vi "SMain.vi"() -> ()   [LabVIEW 2011] (continued)
, 7358893750.0, 7365137500.0, 7371381250.0, 7377625000.0, 7383868750.0, 7390112500.0, 7396356250.0, 7402600000.0, 7408843750.0, 7415087500.0, 7421331250.0, 7427575000.0, 7433818750.0, 7440062500.0, 7446306250.0, 7452550000.0, 7458793750.0, 7465037500.0, 7471281250.0, 7477525000.0, 7483768750.0, 7490012500.0, 7496256250.0, 7502500000.0, 7508743750.0, 7514987500.0, 7521231250.0, 7527475000.0, 7533718750.0, 7539962500.0, 7546206250.0, 7552450000.0, 7558693750.0, 7564937500.0, 7571181250.0, 7577425000.0, 7583668750.0, 7589912500.0, 7596156250.0, 7602400000.0, 7608643750.0, 7614887500.0, 7621131250.0, 7627375000.0, 7633618750.0, 7639862500.0, 7646106250.0, 7652350000.0, 7658593750.0, 7664837500.0, 7671081250.0, 7677325000.0, 7683568750.0, 7689812500.0, 7696056250.0, 7702300000.0, 7708543750.0, 7714787500.0, 7721031250.0, 7727275000.0, 7733518750.0, 7739762500.0, 7746006250.0, 7752250000.0, 7758493750.0, 7764737500.0, 7770981250.0, 7777225000.0, 7783468750.0, 7789712500.0, 7795956250.0, 7802200000.0, 7808443750.0, 7814687500.0, 7820931250.0, 7827175000.0, 7833418750.0, 7839662500.0, 7845906250.0, 7852150000.0, 7858393750.0, 7864637500.0, 7870881250.0, 7877125000.0, 7883368750.0, 7889612500.0, 7895856250.0, 7902100000.0, 7908343750.0, 7914587500.0, 7920831250.0, 7927075000.0, 7933318750.0, 7939562500.0, 7945806250.0, 7952050000.0, 7958293750.0, 7964537500.0, 7970781250.0, 7977025000.0, 7983268750.0, 7989512500.0, 7995756250.0, 8002000000.0, 8008243750.0, 8014487500.0, 8020731250.0, 8026975000.0, 8033218750.0, 8039462500.0, 8045706250.0, 8051950000.0, 8058193750.0, 8064437500.0, 8070681250.0, 8076925000.0, 8083168750.0, 8089412500.0, 8095656250.0, 8101900000.0, 8108143750.0, 8114387500.0, 8120631250.0, 8126875000.0, 8133118750.0, 8139362500.0, 8145606250.0, 8151850000.0, 8158093750.0, 8164337500.0, 8170581250.0, 8176825000.0, 8183068750.0, 8189312500.0, 8195556250.0, 8201800000.0, 8208043750.0, 8214287500.0, 8220531250.0, 8226775000.0, 8233018750.0, 8239262500.0, 8245506250.0, 8251750000.0, 8257993750.0, 8264237500.0, 8270481250.0, 8276725000.0, 8282968750.0, 8289212500.0, 8295456250.0, 8301700000.0, 8307943750.0, 8314187500.0, 8320431250.0, 8326675000.0, 8332918750.0, 8339162500.0, 8345406250.0, 8351650000.0, 8357893750.0, 8364137500.0, 8370381250.0, 8376625000.0, 8382868750.0, 8389112500.0, 8395356250.0, 8401600000.0, 8407843750.0, 8414087500.0, 8420331250.0, 8426575000.0, 8432818750.0, 8439062500.0, 8445306250.0, 8451550000.0, 8457793750.0, 8464037500.0, 8470281250.0, 8476525000.0, 8482768750.0, 8489012500.0, 8495256250.0, 8501500000.0, 8507743750.0, 8513987500.0, 8520231250.0, 8526475000.0, 8532718750.0, 8538962500.0, 8545206250.0, 8551450000.0, 8557693750.0, 8563937500.0, 8570181250.0, 8576425000.0, 8582668750.0, 8588912500.0, 8595156250.0, 8601400000.0, 8607643750.0, 8613887500.0, 8620131250.0, 8626375000.0, 8632618750.0, 8638862500.0, 8645106250.0, 8651350000.0, 8657593750.0, 8663837500.0, 8670081250.0, 8676325000.0, 8682568750.0, 8688812500.0, 8695056250.0, 8701300000.0, 8707543750.0, 8713787500.0, 8720031250.0, 8726275000.0, 8732518750.0, 8738762500.0, 8745006250.0, 8751250000.0, 8757493750.0, 8763737500.0, 8769981250.0, 8776225000.0, 8782468750.0, 8788712500.0, 8794956250.0, 8801200000.0, 8807443750.0, 8813687500.0, 8819931250.0, 8826175000.0, 8832418750.0, 8838662500.0, 8844906250.0, 8851150000.0, 8857393750.0, 8863637500.0, 8869881250.0, 8876125000.0, 8882368750.0, 8888612500.0, 8894856250.0, 8901100000.0, 8907343750.0, 8913587500.0, 8919831250.0, 8926075000.0, 8932318750.0, 8938562500.0, 8944806250.0, 8951050000.0, 8957293750.0, 8963537500.0, 8969781250.0, 8976025000.0, 8982268750.0, 8988512500.0, 8994756250.0, 9001000000.0, 9007243750.0, 9013487500.0, 9019731250.0, 9025975000.0, 9032218750.0, 9038462500.0, 9044706250.0, 9050950000.0, 9057193750.0, 9063437500.0, 9069681250.0, 9075925000.0, 9082168750.0, 9088412500.0, 9094656250.0, 9100900000.0, 9107143750.0, 9113387500.0, 9119631250.0, 9125875000.0, 9132118750.0, 9138362500.0, 9144606250.0, 9150850000.0, 9157093750.0, 9163337500.0, 9169581250.0, 9175825000.0, 9182068750.0, 9188312500.0, 9194556250.0, 9200800000.0, 9207043750.0, 9213287500.0, 9219531250.0, 9225775000.0, 9232018750.0, 9238262500.0, 9244506250.0, 9250750000.0, 9256993750.0, 9263237500.0, 9269481250.0, 9275725000.0, 9281968750.0, 9288212500.0, 9294456250.0, 9300700000.0, 9306943750.0, 9313187500.0, 9319431250.0, 9325675000.0, 9331918750.0, 9338162500.0, 9344406250.0, 9350650000.0, 9356893750.0, 9363137500.0, 9369381250.0, 9375625000.0, 9381868750.0, 9388112500.0, 9394356250.0, 9400600000.0, 9406843750.0, 9413087500.0, 9419331250.0, 9425575000.0, 9431818750.0, 9438062500.0, 9444306250.0, 9450550000.0, 9456793750.0, 9463037500.0, 9469281250.0, 9475525000.0, 9481768750.0, 9488012500.0, 9494256250.0, 9500500000.0, 9506743750.0, 9512987500.0, 9519231250.0, 9525475000.0, 9531718750.0, 9537962500.0, 9544206250.0, 9550450000.0, 9556693750.0, 9562937500.0, 9569181250.0, 9575425000.0, 9581668750.0, 9587912500.0, 9594156250.0, 9600400000.0, 9606643750.0, 9612887500.0, 9619131250.0, 9625375000.0, 9631618750.0, 9637862500.0, 9644106250.0, 9650350000.0, 9656593750.0, 9662837500.0, 9669081250.0, 9675325000.0, 9681568750.0, 9687812500.0, 9694056250.0, 9700300000.0, 9706543750.0, 9712787500.0, 9719031250.0, 9725275000.0, 9731518750.0, 9737762500.0, 9744006250.0, 9750250000.0, 9756493750.0, 9762737500.0, 9768981250.0, 9775225000.0, 9781468750.0, 9787712500.0, 9793956250.0, 9800200000.0, 9806443750.0, 9812687500.0, 9818931250.0, 9825175000.0, 9831418750.0, 9837662500.0, 9843906250.0, 9850150000.0, 9856393750.0, 9862637500.0, 9868881250.0, 9875125000.0, 9881368750.0, 9887612500.0, 9893856250.0, 9900100000.0, 9906343750.0, 9912587500.0, 9918831250.0, 9925075000.0, 9931318750.0, 9937562500.0, 9943806250.0, 9950050000.0, 9956293750.0, 9962537500.0, 9968781250.0, 9975025000.0, 9981268750.0, 9987512500.0, 9993756250.0, 10000000000.0]
  out "Test Graph":refnum<vi>[](array[refnum])
  out "S-Pair Loop":i32=8
  out "S-Para Item List":string[](array[string])=["SDD21", "SDD11", "SCD22", "SCC11", "SCD21-SDD21", "ILD_15"]
  out "S Item Size":i32=6
  out "Spec Association Col No":string[](array[string])=["1", "2", "3", "4", "5", "6", "7"]
  out "Diff Test Item Name":string[](array[string])=["SDD21", "SDD11", "SCD22", "SCC11", "SCD21-SDD21", "NEXT", "ILD_15"]
  out "FEXT Pair Name":string[](array[string])=["TX2-RX1", "TX3-RX1", "TX4-RX1", "TX1-RX2", "TX3-RX2", "TX4-RX2", "TX1-RX3", "TX2-RX3", "TX4-RX3", "TX1-RX4", "TX2-RX4", "TX3-RX4"]
  out "NEXT Pair Name":string[](array[string])=["TX1-RX1", "TX2-RX1", "TX3-RX1", "TX4-RX1", "TX1-RX2", "TX2-RX2", "TX3-RX2", "TX4-RX2", "TX1-RX3", "TX2-RX3", "TX3-RX3", "TX4-RX3", "TX1-RX4", "TX2-RX4", "TX3-RX4", "TX4-RX4"]
  out "S-para Pair Name":string[](array[string])=["TX1", "RX1", "TX2", "RX2", "TX3", "RX3", "TX4", "RX4"]
  in  "Tab_System":enum32{"Test", "Report", "System", "Other"}(tab)=enum."Report"
  out "Pro Num":i64
  out "MO Num":i64
  out "UseAge":i64
  out "Used":i64
  in  "P/N:":string="L99QF015-SD-R"
  in  "S/N:":string="automatic sn"
  in  "MO:":string="E511D-160900761"
  out "proBar":dbl(slide) scale=0.0..100.0
  in  "Start Test":bool
  in  "Sample Description":string="Des:HW QSFP28 Passive Cable\rCable AWG:30\rLength:1000mm"
  in  "Result":string="Testing..."
  in  "Urgent Stop":bool
  in  "Test Status:":string="ILD_15将会采用与SDD21设定方式进行计算\n将生成精简的XML文件"
  in  "Temperature(℃)":string="163190001"
  in  "Relative Humidity(%)":string="163190001"
  in  "Fixture No":string="163190001"
  in  "Sample #":string="163190001"
  in  "Report No.":string="HF-163190001"
  in  "Applicant:":string
  in  "Approval:":u16(ring) items=["Chenhui Zeng", "Jet Shen"]
  in  "Tester:":u16(ring) items=["Wave Zhang", "Longjun Zhou", "Hui Pan", "Lindsay Gu", "Xiaoyue Xiang", "Fenglian Shi"]
  in  "Report Type:":u16(ring) items=["Excel", "Excel&PDF"]
  in  "Use Counts?":bool
  in  "By Channel?":bool
  out "Dem 2X":bool=TRUE
  in  "Local Database":bool
  in  "Demo":bool=TRUE
  in  "Manual":bool
  in  "Crosstalk  by Trace":bool
  in  "Adaptor:":enum16{"RS232 - IIC", "LUXSHARE - IIC"}(ring)=enum."LUXSHARE - IIC"
  in  "DAQ  Model:":T14(ring)
  in  "VNA VISA":refnum<visa-resource-name>="E5071C"
  in  "VNA Model:":enum16{"E5071C", "N5230A(C)", "N5224A"}(ring)
  in  "Port Type":u16(ring)=1
  in  "DAQ Device":u16(ring) items=["Dev1", "Dev2", "Dev3"]
  in  "Impedance Spec String":string="0.75@110@2@110;0.75@90@2@95"
  in  "VISA COM":refnum<visa-resource-name>="COM4"
  in  "Printer VISA":refnum<visa-resource-name>="COM4"
  in  "RS232 I2C VISA":refnum<visa-resource-name>="COM3"
  in  "save config":bool
  in  "打印模式":enum16{"IT Print", "EE Print"}(ring)=enum."EE Print" caption="Print Mode"
  in  "RS232 I2C Counts":refnum<visa-resource-name>="COM3"
  in  "Auto Count:":bool
  in  "Fast Print":bool=TRUE
  in  "测试模式":u16(ring) items=["正常", "调机", "校正"]
  in  "制程条码":bool
  in  "SN Keep":bool
  in  "Pre Check":bool
  in  "Type":u16(ring) items=["SFP+", "QSFP28"]
  in  "preStation":string="A0075"
  out "Current Testing Label/当前测试条码":string
  out "ratio":dbl format="%#_g%%"
  out "Total":dbl
  out "Failed":dbl
  out "Passed":dbl
  in  "线别":u16(ring) items=["XT026", "XT027", "XT028", "other"]
  in  "sampleNo":u16(ring) items=["0.009", "014-30", "11", "125553", "15669", "2018     8     20", "2018   8  7", "233665", "741", "755", "785587", "7896987", "a", "L021254", "L9956255", "L99901", "L99SF014-SD-H校准", "L99SF025-SD-R", "LDUQF007-18.6.22", "校准"]
  in  "Tab_Graph":T15(tab)
  out "PASS":cluster{"Horz Time array":dbl[], "Y":dbl[]}[](graph) caption="SDD21"
  out "PASS":cluster{"Horz Time array":dbl[], "Y":dbl[]}[](graph) caption="SDD11"
  out "Test Graph3":cluster{"Horz Time array":dbl[], "Y":dbl[]}[](graph) caption="SCC11"
  out "Test Graph4":cluster{"Horz Time array":dbl[], "Y":dbl[]}[](graph) caption="SCD21-SDD21"
  out "Test Graph5":cluster{"Horz Time array":dbl[], "Y":dbl[]}[](graph) caption="ILD"
  out "Test Graph6":cluster{"Horz Time array":dbl[], "Y":dbl[]}[](graph) caption="ILD"
  out "Test Graph7":cluster{"Horz Time array":dbl[], "Y":dbl[]}[](graph) caption="SCD21-SDD21"
  out "Test Graph8":cluster{"Horz Time array":dbl[], "Y":dbl[]}[](graph) caption="Pskew"
  out "TDD11 Graph":cluster{"Horz Time array":dbl[], "Y":dbl[]}[](graph) caption="TDD11"
  out "TDD22 Graph":cluster{"Horz Time array":dbl[], "Y":dbl[]}[](graph) caption="TDD22"
  out "TCC11":cluster{"Horz Time array":dbl[], "Y":dbl[]}[](graph) caption="TDD22"
  out "TCC22":cluster{"Horz Time array":dbl[], "Y":dbl[]}[](graph) caption="TDD22"
  out "Delay":cluster{"Horz Time array":dbl[], "Y":dbl[]}[](graph) caption="TDD22"
  out "Next":cluster{"Horz Time array":dbl[], "Y":dbl[]}[](graph) caption="NEXT"
  out "Test Graph10":cluster{"Horz Time array":dbl[], "Y":dbl[]}[](graph) caption="FEXT_TX2-RX1"
  out "MDFEXT":cluster{"Horz Time array":dbl[], "Y":dbl[]}[](graph) caption="FEXT_TX2-RX1"
  out "MDNEXT":cluster{"Horz Time array":dbl[], "Y":dbl[]}[](graph) caption="FEXT_TX2-RX1"
  # "HPTS Of  VNA Automatic Measurement System"
  # "Rev: 3.0.0.0\n18/06/07"
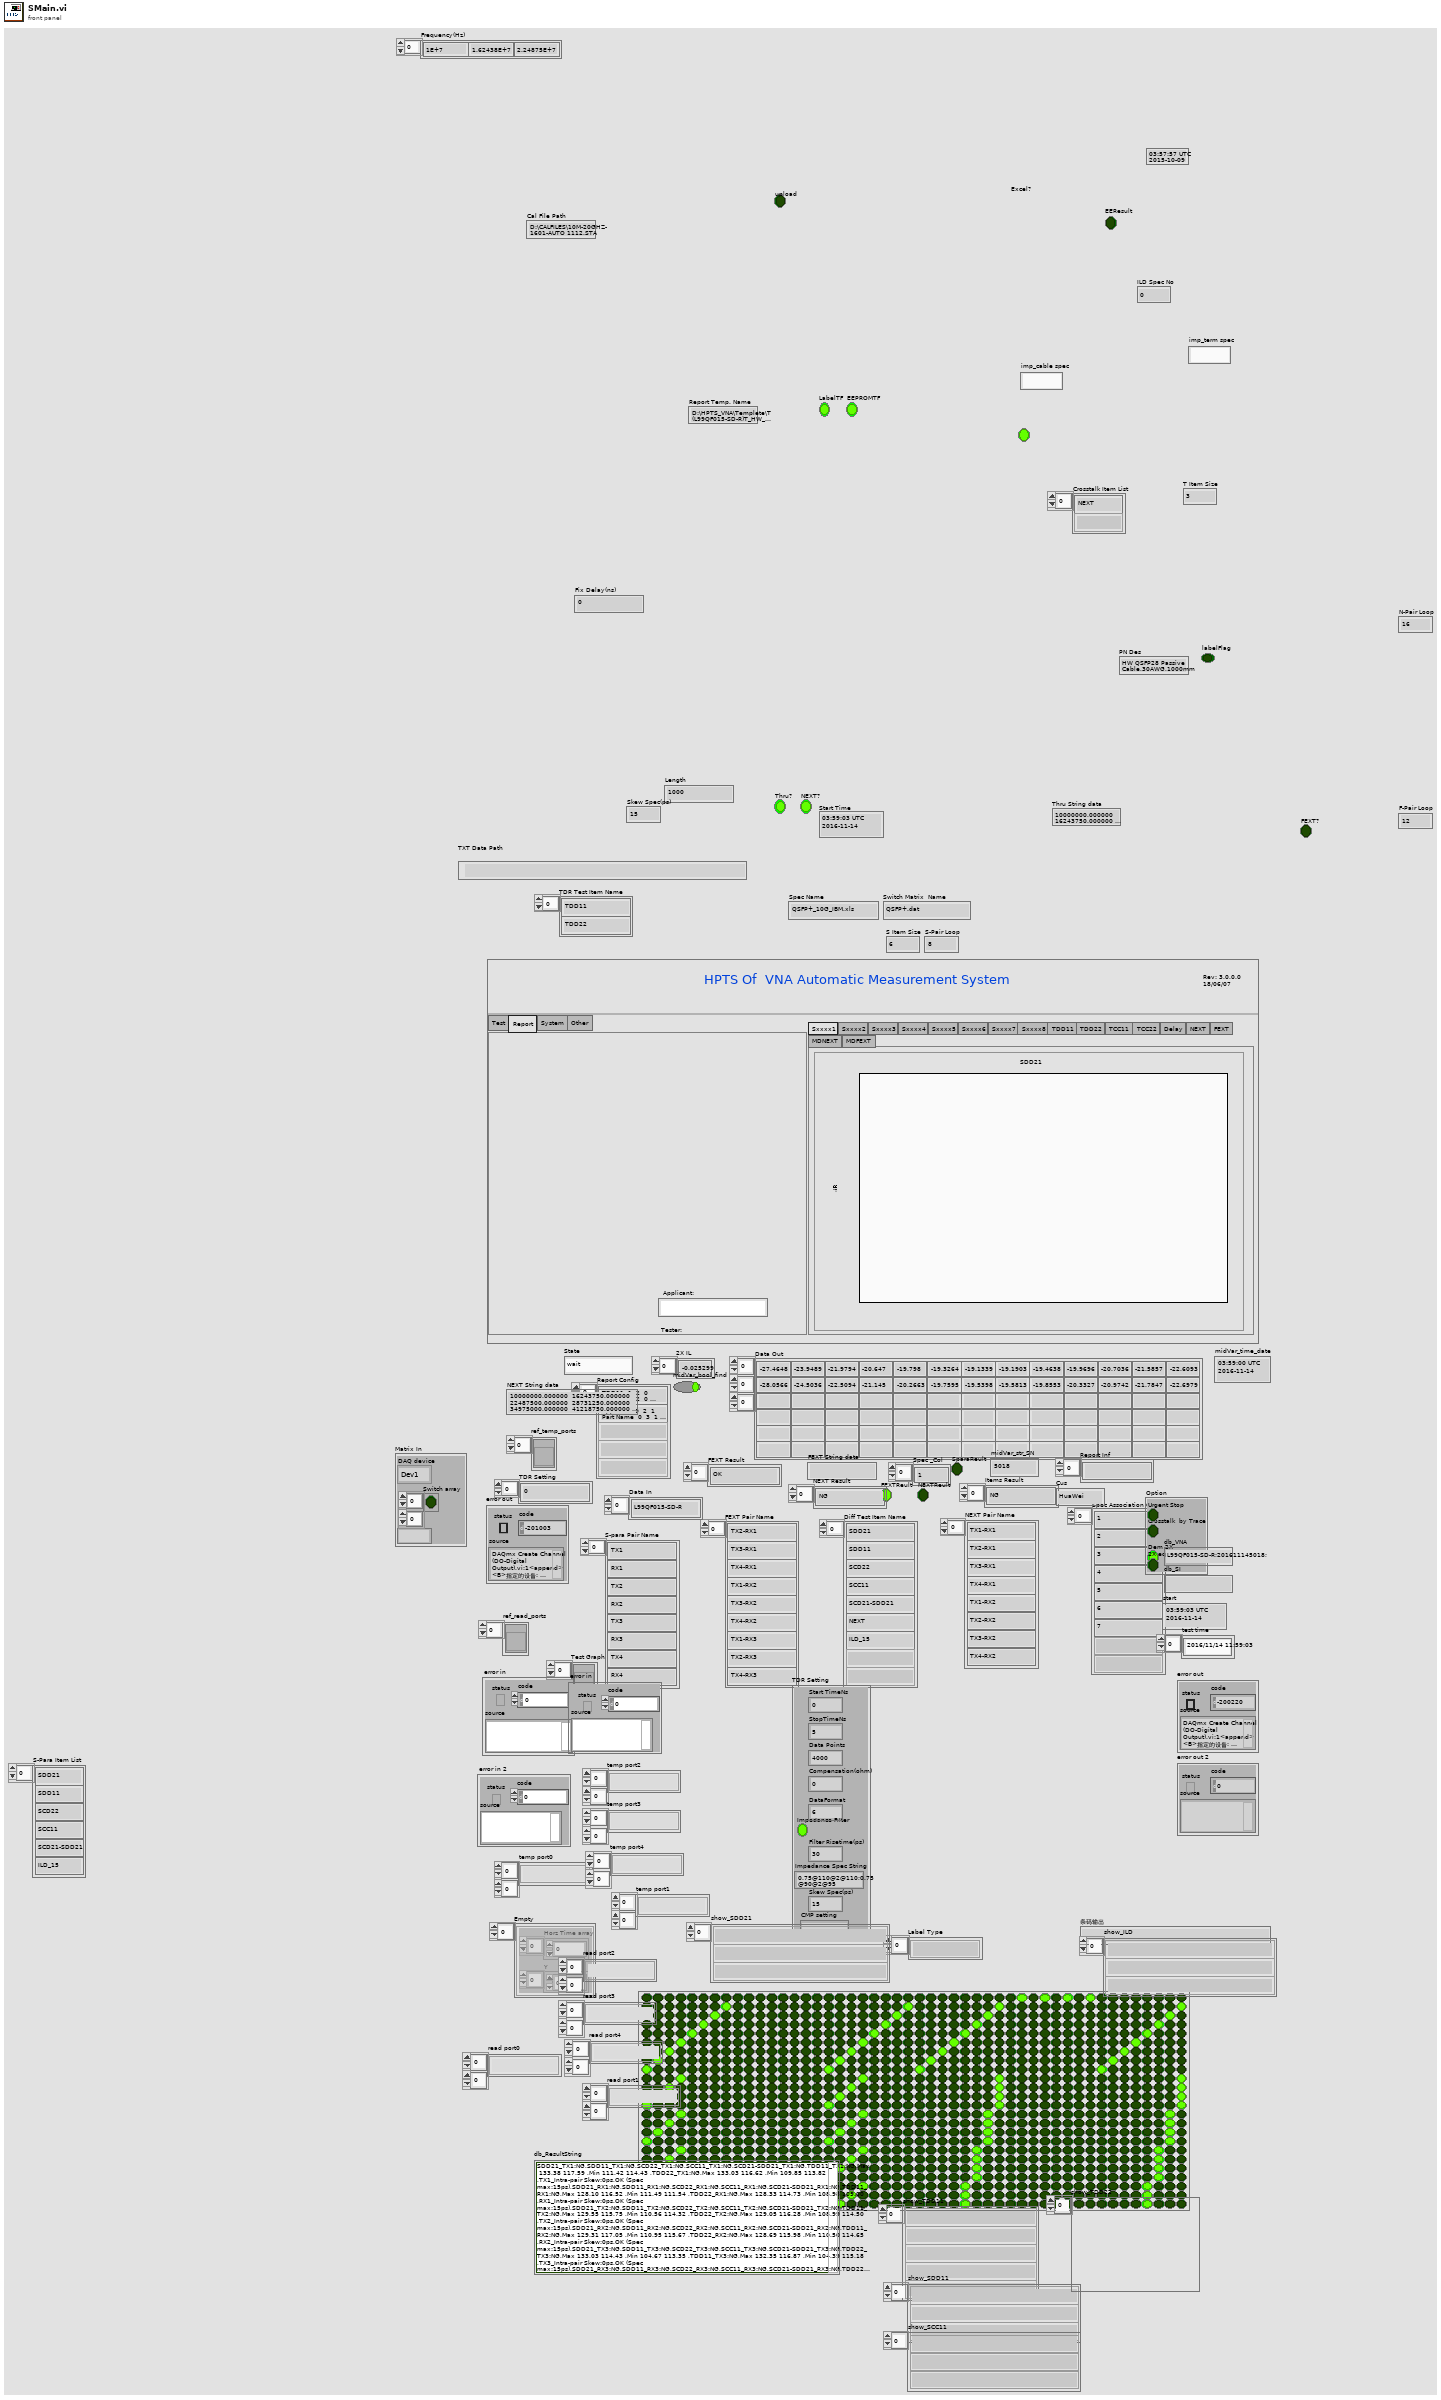
[diagram p1: front panel]
types:
  T1 = typedef "UploadPara.ctl" = cluster{"NetCmdHW":string, "NetPathHW":string, "NetCmdCompress":string, "NetPathCompress1":string, "NetPathCompress2":string, "AlarmDisplay":string, "Synchronous":string, "NetTemppath":string, "NetLocalpath":string}
  T2 = typedef "cluResult.ctl" = cluster{"itemResult":string[], "itemName":string[]}
  T3 = typedef "singleTestParameter.ctl" = cluster{"itemName":string, "testPair":dbl, "chartDisplay?":bool, "spec":cluster{"upper limit":cluster{"dx":dbl[], "dy":dbl[]}, "lowwer limit":cluster{"dx":dbl[], "dy":dbl[]}}, "smooth":cluster{"smooth?":bool, "smoothPoints":dbl}, "Compensation(ohm)":dbl, "Filter Risetime(ps)":dbl, "singlePoint":string[], "offset":dbl[]}
  T4 = typedef "informationIn.ctl" = cluster{"Sample PN: ":string, "SampleSN:":string, "Sparam Test Item":string[], "S-para Pair Name":string[], "Length":string, "Diff Test Item Name":string[], "Diff Test Item Name smooth":string[], "smooth point":dbl, "limitSpec":string[][], "switchIndexOffset":i32, "testType":enum16{"Loss", "Next", "Fext"}, "pairStartIndex":i32, "DAQ  Model:":enum16{"NI PCI-6509", "LX MCU", "LX MCU_40G", "LX MCU_40G_HuaWei"}, "VISA COM":refnum<visa-resource-name>, "Matrix  In":bool[][]}
  T5 = cluster{"Tab_Graph":refnum<vi>, "Test Graph":refnum<vi>[], "Test Status:":refnum<vi>, "db_ResultString":refnum<vi>}
  T6 = cluster{"Start TimeNs":dbl, "StopTimeNs":dbl, "Data Points":i32, "Compensation(ohm)":dbl, "DataFormat":i16, "Impedance Filter":bool, "Filter Risetime(ps)":dbl, "Impedance Spec String":string, "Skew Spec(ps)":i32, "CMP Setting":string}[]
  T7 = cluster{"start":i32, "length":i32, "p":i32, "H/L":bool}[]
  T8 = cluster{"Server":string, "DB":string, "PSW":string, "User":string}
  T9 = cluster{"auto get refer point":bool, "width1":i32, "width2":i32, "show_TDD11":string[], "show_TDD22":string[], "test time":string[], "show_impspec":string[], "TestResult":bool[], "FileName":string, "FileVersion":string}
  T10 = cluster{"Start TimeNs":dbl, "StopTimeNs":dbl, "Data Points":i32, "Compensation(ohm)":dbl, "DataFormat":i16, "Impedance Filter":bool, "Filter Risetime(ps)":dbl, "Impedance Spec String":string, "Skew Spec(ps)":i32, "CMP Setting":string}
  T11 = cluster{"Urgent Stop":bool, "Crosstalk  by Trace":bool, "Dem 2X":bool, "2X equalize ":bool}
  T12 = cluster{"Start TimeNs":dbl, "StopTimeNs":dbl, "Data Points":i32, "Compensation(ohm)":dbl, "DataFormat":i16, "Impedance Filter":bool, "Filter Risetime(ps)":dbl, "Impedance Spec String":string, "Skew Spec(ps)":i32, "CMP setting":string}
  T13 = cluster{"DAQ device":enum16{"Dev1", "Dev2", "Dev3"}, "Switch array ":bool[][], i32}
  T14 = enum16{"NI PCI-6509", "LX MCU", "LX MCU_40G", "LX MCU_40G_HuaWei"}
  T15 = enum32{"Sxxxx1", "Sxxxx2", "Sxxxx3", "Sxxxx4", "Sxxxx5", "Sxxxx6", "Sxxxx7", "Sxxxx8", "TDD11", "TDD22", "TCC11", "TCC22", "Delay", "NEXT", "FEXT", "MDNEXT", "MDFEXT"}
  T16 = enum16{"Standard Report", "HTML", "Word", "Excel"}
  T17 = enum8{"Enabled", "Disabled", "Disabled and Grayed Out"}
  T18 = typedef "HW_xml.ctl" = cluster{"FileVersion":string, "FileName":string, "test time":string[], "original Path":path, "show_impspec":string[], "usedSN":string, "show_Terminal Point":dbl[], "show_Cable Point":dbl[], "sSpec":T3[], "resultCluster":T2, "customerPN":string}
  T19 = enum32{"invalid app kind", "Development System", "Run Time System", "Student Edition", "Embedded LabVIEW", "Evaluation", "Custom"}
  T20 = cluster{"Urgent Stop":bool, "Crosstalk  by Trace":bool, "Dem 2X":bool, "2x equalize ":bool}
  T21 = cluster{"Demo":bool, "Manual":bool, "Urgent Stop":bool}
  T22 = cluster{"DAQ Device":u16, "Switch array ":bool[][], i32}
  T23 = cluster{"Start TimeNs 2":dbl, "StopTimeNs 2":dbl, "Data Points 2":i32, "Compensation(ohm) 2":dbl, "DataFormat":i16, bool, "Filter Risetime(ps) 2":dbl, "Impedance Spec String 2":string, "Skew Spec(ps) 2":i32, string}
  T24 = cluster{"DAQ Device":u16, "Switch array ":bool[][], "S-Pair Loop":i32}
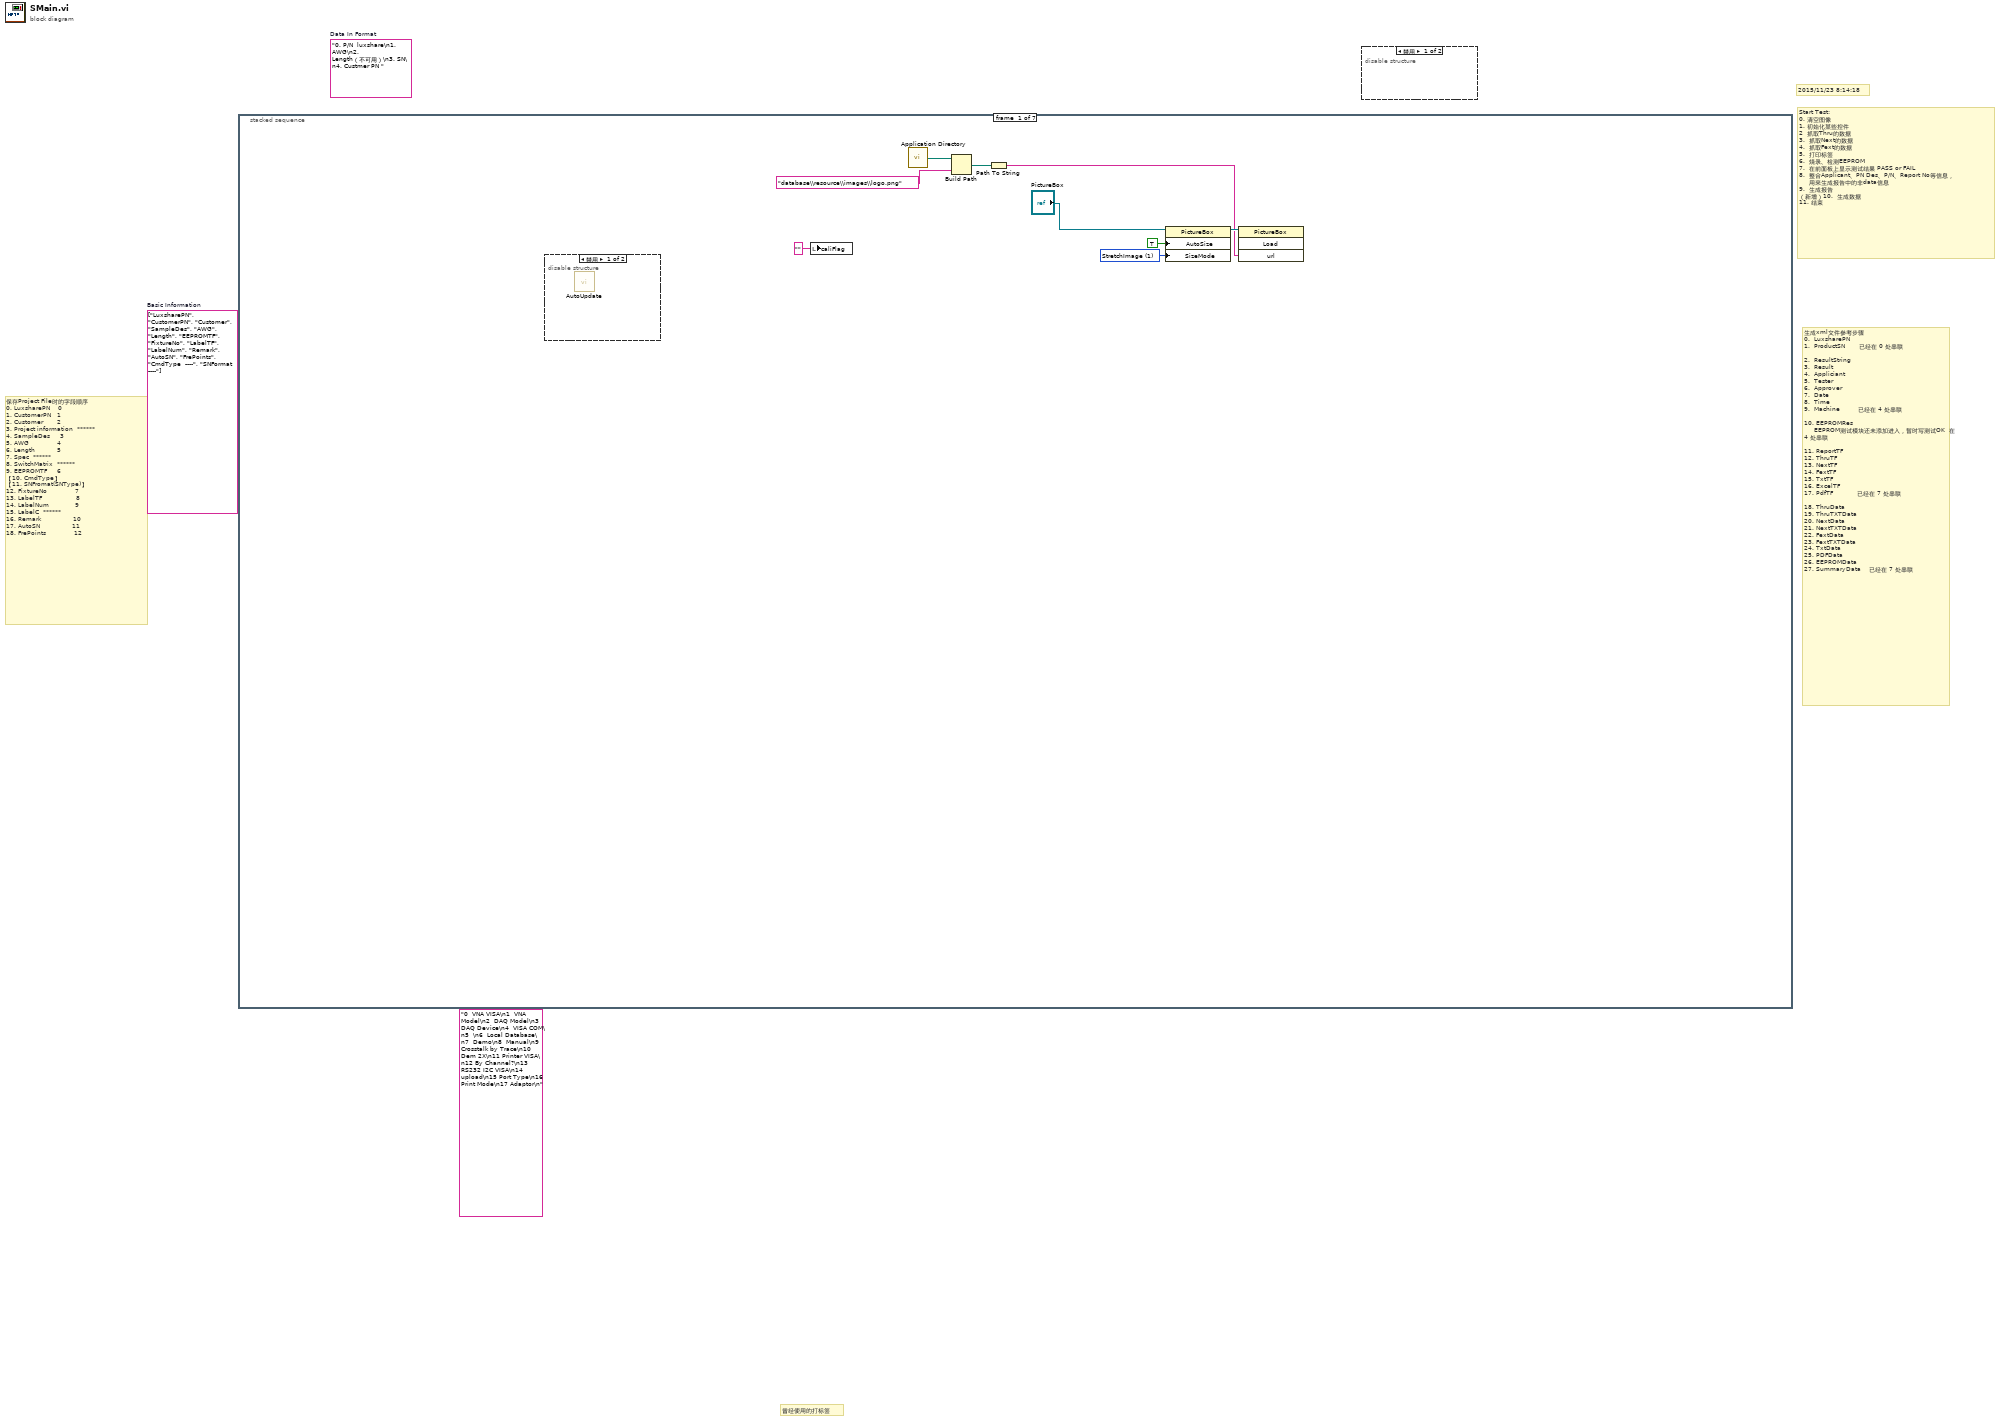
[diagram p0: block diagram]
diagram:
  (unwired) "0  VNA VISA\n1  VNA Model\n2  DAQ Model\n3  DAQ Device\n4  VISA COM\n5  \n6  Local Database\n7  Demo\n8  Manual\n9  Crosstalk by Trace\n10 Dem 2X\n11 Printer VISA\n12 By Channel?\n13 RS232 I2C VISA\n14 upload\n15 Port Type\n16 Print Mode\n17 Adaptor\n"
  (unwired) string[] ["LuxsharePN", "CustomerPN", "Customer", "SampleDes", "AWG", "Length", "EEPROMTF", "FixtureNo", "LabelTF", "LabelNum", "Remark", "AutoSN", "FrePoints", "CmdType  ----", "SNFormat ----"]  # Basic Information
  (unwired) "0. P/N  luxshare\n1. AWG\n2. Length（不可用）\n3. SN\n4. Custmer PN "  # Data In Format
  # "曾经使用的打标签"
  # "保存Project File时的字段顺序\n0. LuxsharePN    0 \n1. CustomerPN   1\n2. Customer       2\n3. Project information  ****** \n4. SampleDes     3\n5. AWG              4\n6. Length           5\n7. Spec  ******\n8. SwitchMatrix  ******  \n9. EEPROMTF     6\n【10. CmdType】           \n【11. SNFromat(SNType)】   \n12. FixtureNo              7\n13. LabelTF                 8\n14. LabelNum             9\n15. LabelC  ******\n16. Remark                10\n17. AutoSN                11\n18. FrePoints              12"
  # "2015/11/23 8:14:18"
  # "生成xml文件参考步骤\n0.  LuxsharePN\n1.  ProductSN       已经在 0 处串联\n\n2.  ResultString     \n3.  Result             \n4.  Appliciant\n5.  Tester\n6.  Approver\n7.  Date \n8.  Time\n9.  Machine         已经在 4 处串联\n\n10. EEPROMRes   \n     EEPROM测试模块还未添加进入，暂时写测试OK  在 4 处串联\n\n11. ReportTF\n12. ThruTF\n13. NextTF\n14. FextTF\n15. TxtTF\n16. ExcelTF\n17. PdfTF            已经在 7 处串联\n\n18. ThruData\n19. ThruTXTData\n20. NextData\n21. NextTXTData\n22. FextData\n23. FextTXTData\n24. TxtData\n25. PDFData\n26. EEPROMData\n27. SummaryData    已经在 7 处串联"
  # "Start Test:\n0. 清空图像\n1. 初始化某些控件 \n2  抓取Thru的数据\n3.  抓取Next的数据\n4.  抓取Fext的数据\n5.  打印标签\n6.  烧录、检测EEPROM\n7.  在前面板上显示测试结果 PASS or FAIL\n8.  整合Applicant、PN Des、P/N、Report No等信息，\n     用来生成报告中的非data信息\n9.  生成报告\n（新增）10.  生成数据 \n11. 结束"
  n1 = stacked-sequence {
    frame #0 {
      w5 = 1 items=["Normal", "StretchImage", "AutoSize", "CenterImage", "Zoom"] ("SizeMode")
      n2 = disable-structure shown="禁用" {
        frame Disabled {
          n3 = call "AutoUpdate.vi"() -> ()  [unwired: 8 in, 2 out]
        }
        frame Enabled {
        }
      }
      n4 = local write "caliFlag"("" ("caliFlag")) -> ()
      n5 = call <vilib>:"Application Directory.vi"() -> ("Application Directory"=w4:path)
      n6 = Build Path(base path=w4, name or relative path="database\\resource\\images\\logo.png" ("名称或相对路径")) -> (appended path=w2:path)
      n7 = Path To String(path=w2) -> (string=w1:string)
      n8 = property class="PictureBox"(reference="PictureBox", "AutoSize"=TRUE, "SizeMode"=w5) -> (reference out=w7:refnum<k24>)  [unwired: 1 in, 1 out]
      n9 = invoke class="PictureBox" method="Load"(reference=w7, "url"=w1) -> ()  [unwired: 2 in, 4 out]
    }
    frame #1 {
      # "中间变量"
      n10 = property class="App"() -> ("App.Kind"=w10:T19)  [unwired: 2 in, 2 out]
      n11 = case shown="\"Run Time System\", 默认" w10 {
        frame "Run Time System", Default {
          w12 = ".exe" ("正则表达式")
          n12 = Current VI's Path() -> (path=w15:path)
          n13 = Path To String(path=w15) -> (string=w14:string)
          n14 = xnode "匹配正则表达式"("输入字符串"=w14, "正则表达式"=w12) -> ("匹配之前"=w13:string)  [unwired: 4 in, 4 out]
          n15 = call <vilib>:"Application Directory.vi"() -> ("Application Directory"=w25:path)
          n16 = Build Path(base path=w25, name or relative path="AutoUpdate.xml" ("名称或相对路径")) -> (appended path=w23:path)
          n17 = Concatenate Strings(w13, w12) -> (→"FileName":string)
          n18 = call "xmlConfigRead.vi"("path to XML document"=w23, "XPath expression"="//@Ver") -> ("OutParaArray"=w22:string[])  [unwired: 2 out]
          n19 = Index Array(array=w22, index=4 ("索引")) -> (element=w17:string)
          n20 = call <vilib>:"Trim Whitespace.vi"("string"=w17) -> ("trimmed string"=w20:string)  [unwired: 1 in]
          n21 = String Length(string=w20) -> (length=w19:i32)
          n22 = Equal To 0?(x=w19) -> (x = 0?=w18:bool)
          n23 = case shown="假" w18 {
            tunnel: w17 -> [w138 _]
            tunnel: [w138 "9.9.9.9" ("node text")] -> w16
            frame False {
            }
            frame True {
              n24 = One Button Dialog(message="读取AutoUpdate.xml失败，使用程序默认版本号9.9.9.9" ("消息")) -> ()  [unwired: 1 in, 1 out]
            }
          }
          "FileVersion" <- w16
        }
        frame "Development System" {
          w141 = "DevelopmentSystem" ("FileName")
          n25 = property on="FileName" class="Str"("Value"=w141) -> ()  [unwired: 2 in, 2 out]
          n26 = property on="FileVersion" class="Str"("Value"=w141) -> ()  [unwired: 2 in, 2 out]
        }
      }
    }
    frame #2 {
      w160 = u16 0 items=["Excel", "Excel&PDF"] ("Report Type:")
      w161 = FALSE ("可见")
      w157 = FALSE ("Manual")
      w202 = 2 ("索引")
      w169 = "" ("Sample Description")
      w204 = 0 ("索引")
      n27 = control-ref of="proBar"() -> (→"proBar_ref":refnum<vi>)
      n28 = local write "preStation"("" ("preStation")) -> ()
      n29 = local write "Excel?"(FALSE ("Local Database")) -> ()
      n30 = local write "AutoSN"(FALSE ("AutoSN")) -> ()
      n31 = local write "P/N:"(w169) -> ()
      n32 = property on="Sample Description" class="Str"("Value"="" ("Sample Description"), "Visible"=FALSE ("可见")) -> ()  [unwired: 2 in, 2 out]
      n33 = property on="Tab_System" class="TabCtl (严格)"("Value"=w204) -> ()  [unwired: 2 in, 2 out]
      n34 = property on="Tab_Graph" class="TabCtl (严格)"("Value"=w204) -> ()  [unwired: 2 in, 2 out]
      n35 = property on="Start Test" class="Bool"("DisabledEnum"=w202) -> ()  [unwired: 2 in, 2 out]
      n36 = property on="VNA Initial" class="Bool"("DisabledEnum"=w202) -> ()  [unwired: 2 in, 2 out]
      n37 = local write "Impedance Spec String"(w169) -> ()
      n38 = control-ref of="Delay"() -> (w142:refnum<vi>)
      n39 = control-ref of="TCC11"() -> (w144:refnum<vi>)
      n40 = control-ref of="TCC22"() -> (w143:refnum<vi>)
      n41 = local write "State"("wait" ("state")) -> ()
      n42 = control-ref of="MDNEXT"() -> (w145:refnum<vi>)
      n43 = control-ref of="PASS"() -> (w214:refnum<vi>)
      n44 = control-ref of="PASS"() -> (w213:refnum<vi>)
      n45 = control-ref of="Test Graph3"() -> (w212:refnum<vi>)
      n46 = control-ref of="Test Graph4"() -> (w211:refnum<vi>)
      n47 = control-ref of="Test Graph5"() -> (w210:refnum<vi>)
      n48 = control-ref of="Test Graph6"() -> (w209:refnum<vi>)
      n49 = control-ref of="Test Graph7"() -> (w208:refnum<vi>)
      n50 = control-ref of="Test Graph8"() -> (w207:refnum<vi>)
      n51 = control-ref of="TDD11 Graph"() -> (w194:refnum<vi>)
      n52 = control-ref of="TDD22 Graph"() -> (w193:refnum<vi>)
      n53 = control-ref of="Next"() -> (w192:refnum<vi>)
      n54 = control-ref of="Test Graph10"() -> (w191:refnum<vi>)
      n55 = control-ref of="MDFEXT"() -> (w146:refnum<vi>)
      n56 = local write "Current Testing Label/当前测试条码"("") -> ()
      n57 = Build Array(w214, w213, w212, w211, w210, w209, w208, w207, w194, w193, w144, w143, w142, w192, w191, w146, w145) -> (w206:refnum<vi>[])
      "Test Graph" <- w206
      n58 = property on="Result" class="Str"("Visible"=FALSE ("可见"), "Value"="Testing..." ("Result"), "DisabledEnum"=1, "Text.BGColor"=u32 16777216) -> ()  [unwired: 2 in, 2 out]
      n59 = local write "Demo"(w157) -> ()
      n60 = local write "Dem 2X"(w157) -> ()
      n61 = local write "Manual"(w157) -> ()
      n62 = local write "Excel?"(w157) -> ()
      n63 = property on="Urgent Stop" class="Bool (严格)"("DisabledEnum"=0 ("索引")) -> ()  [unwired: 2 in, 2 out]
      n64 = property on="Report Type:" class="Ring (严格)"("Value"=w160) -> ()  [unwired: 2 in, 2 out]
      n65 = property on="Start Page" class="DigNum (严格)"("Visible"=w161) -> ()  [unwired: 2 in, 2 out]
      n66 = property on="End Page" class="DigNum (严格)"("Visible"=w161) -> ()  [unwired: 2 in, 2 out]
      n67 = local write "Local Database"(w157) -> ()
      n68 = local write "Auto Count:"(w157) -> ()
      n69 = local write "Crosstalk  by Trace"(w157) -> ()
      n70 = local write "Urgent Stop"(w157) -> ()
      n71 = for {
        tunnel: w206 -> [w248] mode=indexing
        tunnel: "Empty" -> [w247]
        n72 = property class="XYGraph (严格)"(reference=w248, "Value"=w247, "Caption.Visible"=FALSE ("标题.可见")) -> ()  [unwired: 1 in, 2 out]
      }
      n73 = call "运行批处理.vi"() -> ()  [unwired: 12 in]
      n74 = local write "Use Counts?"(TRUE ("Use Counts?")) -> ()
      n75 = local read "VISA COM"() -> (w168:refnum<visa-resource-name>)
      n76 = local read "DAQ Device"() -> (w166:u16)
      n77 = stacked-sequence {
        frame #0 {
          n78 = control-ref of="temp port0"() -> (w220:refnum<vi>)
          n79 = control-ref of="temp port1"() -> (w219:refnum<vi>)
          n80 = control-ref of="temp port2"() -> (w218:refnum<vi>)
          n81 = control-ref of="temp port3"() -> (w217:refnum<vi>)
          n82 = control-ref of="temp port4"() -> (w216:refnum<vi>)
          n83 = Build Array(w220, w219, w218, w217, w216) -> (→"ref_temp_ports":refnum<vi>[])
        }
        frame #1 {
          n84 = control-ref of="read port0"() -> (w226:refnum<vi>)
          n85 = control-ref of="read port1"() -> (w225:refnum<vi>)
          n86 = control-ref of="read port2"() -> (w224:refnum<vi>)
          n87 = control-ref of="read port3"() -> (w223:refnum<vi>)
          n88 = control-ref of="read port4"() -> (w222:refnum<vi>)
          n89 = Build Array(w226, w225, w224, w223, w222) -> (→"ref_read_ports":refnum<vi>[])
        }
      }
      n90 = local read "Manual"() -> (w164:bool)
      n91 = local read "DAQ  Model:"() -> (w167:T14)
      n92 = local read "Demo"() -> (w163:bool)
      n93 = Format Date/Time String(time format string (%c)="%#j") -> (date/time string=w197:string)  [unwired: 2 in]
      n94 = String Length(string=w197) -> (length=w198:i32)
      n95 = Or(x=w164, y=w163) -> (x .or. y?=w165:bool)
      n96 = call <vilib>:"Application Directory.vi"() -> ("Application Directory"=w181:path)
      n97 = case shown="2" w198 {
        tunnel: w197 -> [w240 w244 w245]
        tunnel: [w239 w243 w245] -> w196
        frame 1, Default {
          n98 = Concatenate Strings("00" ("字符串"), w240) -> (w239:string)
        }
        frame 2 {
          n99 = Concatenate Strings("0" ("字符串"), w244) -> (w243:string)
        }
        frame 3 {
        }
      }
      n100 = Build Path(base path=w181, name or relative path="database\\inf.txt" ("名称或相对路径")) -> (appended path=w179:path)
      n101 = case shown="假" w165 {
        tunnel: w166 -> [w229 _]
        tunnel: w167 -> [w228 _]
        tunnel: w168 -> [w227 _]
        frame False {
          n102 = case shown="\"LX MCU\"" w228 {
            tunnel: w229 -> [w234 _ _]
            tunnel: w227 -> [_ w236 w238]
            frame "NI PCI-6509", Default {
              n103 = local read "Switch array"() -> (w232:bool[][])
              n104 = call "6509 simple.vi"("error in"="error in", "index (row)"=i8 79, "array input: P0-P1-P2-P3-P4-P5"=w232, "DAQ device"=w234) -> ("error out"=→"error out":errorcluster)  [unwired: 3 in]
            }
            frame "LX MCU" {
              w235 = u16 1 items=["Testing", "Close All"] ("Function")
              n105 = call "MCU Switch Control.vi"("Function"=w235, "VISA"=w236) -> ()  [unwired: 9 in, 1 out]
            }
            frame "LX MCU_40G" {
              w237 = u16 1 items=["Testing", "Close All"] ("Function")
              n106 = call "40G MCU Switch Control.vi"("Function"=w237, "VISA"=w238) -> ()  [unwired: 9 in, 1 out]
            }
          }
        }
        frame True {
        }
      }
      n107 = call-poly <vilib>:"Read From Spreadsheet File.vi"("file path (dialog if empty)"=w179) -> ("all rows"=w178:string[][])  [unwired: 6 in, 4 out]
      n108 = Delete From Array(array=w178, index (row)=0 ("索引 (行)")) -> (array with subset deleted=w176:string[][])  [unwired: 2 in, 1 out]
      n109 = Format Date/Time String(time format string (%c)="%#y") -> (date/time string=w201:string)  [unwired: 2 in]
      n110 = Index Array(array=w176, index (col) #1=6 ("禁用的索引 (列)"), index (col) #2=7 ("索引 (列)")) -> (element #1=w173:string[], element #2=w172:string[])  [unwired: 2 in]
      n111 = Concatenate Strings(w201, w196, "0001" ("字符串")) -> (w182:string)
      n112 = call "Delete empty element from array.vi"("Array In"=w173) -> ("Array out"=w171:string[])  [unwired: 26 in]
      n113 = local write "Sample #"(w182) -> ()
      n114 = call "Delete empty element from array.vi"("Array In"=w172) -> ("Array out"=w170:string[])  [unwired: 26 in]
      n115 = local write "S/N:"(w182) -> ()
      n116 = Concatenate Strings("HF-" ("字符串"), w182) -> (w184:string)
      n117 = property on="Approval:" class="Ring (严格)"("Strings []"=w170) -> ()  [unwired: 2 in, 2 out]
      n118 = property on="Tester:" class="Ring (严格)"("Strings []"=w171) -> ()  [unwired: 2 in, 2 out]
      n119 = local write "Test Status:"("Please do full calibration for VNA with E-Cal module before start test!\nThen, click \"VNA initial\" buttom to recall calibration file!" ("Test Status:")) -> ()
      n120 = local write "Report No."(w184) -> ()
      "proBar" <- u8 0 ("proBar")
      "Go" <- FALSE ("show_bool_checkResult")
      "UseAge" <- u8 0 ("寿命")
      "Used" <- u8 0 ("已用")
      "strFSN 原始SN" <- "" ("strFSN 原始SN")
    }
    frame #3 {
      (unwired) string[][] [["VNA VISA", "E5071C"], ["VNA Model", "E5071C"], ["DAQ Model", "NI PCI-6509"], ["DAQ Device", "Dev1"], ["VISA COM", "COM4"], ["checkBeforeTest", "FALSE"], ["Local Database", "TRUE"], ["Demo", "TRUE"], ["Manual", "FALSE"], ["Crosstalk by Trace", "FALSE"], ["Dem 2X", "FALSE"], ["By Channel?", "FALSE"], ["Print VISA", "USB0::0x0A5F::0x00AB::JJL045601::RAW"], ["RS232 I2C VISA", "COM1"], ["Data UpLoad", "FALSE"], ["Port Type", "1"], ["Print Mode", "IT Print"], ["Adaptor", "RS232 - IIC"]] ("all rows")
      (unwired) "0  VNA VISA\n1  VNA Model\n2  DAQ Model\n3  DAQ Device\n4  VISA COM\n5  \n6  Local Database\n7  Demo\n8  Manual\n9  Crosstalk by Trace\n10 Dem 2X\n11 Printer VISA\n12 By Channel?\n13 RS232 I2C VISA\n14 upload\n15 Port Type\n16 Print Mode\n17 Adaptor\n"
      # "加载主页面配置信息"
      n121 = call <vilib>:"Application Directory.vi"() -> ("Application Directory"=w253:path)
      n122 = Build Path(base path=w253, name or relative path="database\\initializeConfig.txt" ("名称或相对路径")) -> (appended path=w251:path)
      n123 = call <vilib>:"Check if File or Folder Exists.vi"("path"=w251) -> ("file or folder exists?"=w250:bool, "dup path"=w249:path)  [unwired: 8 in, 1 out]
      n124 = case shown="真" w250 {
        tunnel: w249 -> [w315 w353]
        frame False {
          w259 = string[][] [["VNA VISA", "E5071C"], ["VNA Model", "E5071C"], ["DAQ Model", "NI PCI-6509"], ["DAQ Device", "Dev1"], ["VISA COM", "COM4"], ["checkBeforeTest", "FALSE"], ["Local Database", "TRUE"], ["Demo", "TRUE"], ["Manual", "FALSE"], ["Crosstalk by Trace", "FALSE"], ["Dem 2X", "FALSE"], ["By Channel?", "FALSE"], ["Print VISA", "USB0::0x0A5F::0x00AB::JJL045601::RAW"], ["RS232 I2C VISA", "COM1"], ["Data UpLoad", "FALSE"], ["Port Type", "1"], ["Print Mode", "IT Print"], ["Adaptor", "RS232 - IIC"], ["Use Counts", "TRUE"], ["RS232 I2C VISA Counts", "COM1"]] ("all rows")
          n125 = Index Array(array=w259, index (col)=1 ("禁用的索引 (列)")) -> (element=w269:string[])  [unwired: 1 in]
          n126 = call-poly <vilib>:"Write To Spreadsheet File.vi"("2D data"=w259, "file path (dialog if empty)"=w315) -> ()  [unwired: 6 in, 1 out]
          n127 = Index Array(array=w269, index #1=0 ("索引"), index #6=5 ("索引"), index #11=10 ("索引"), index #16=15 ("索引")) -> (element #1=w276:string, element #2=w314:string, element #3=w312:string, element #4=w310:string, element #5=w309:string, element #6=w301:string, element #7=w300:string, element #8=w293:string, element #9=w289:string, element #10=w285:string, element #11=w283:string, element #12=w279:string, element #13=w278:string, element #14=w277:string, element #15=w272:string, element #16=w265:string, element #17=w263:string, element #18=w260:string, element #19=w256:string, element #20=w254:string)  [unwired: 16 in]
          n128 = local write "RS232 I2C Counts"(w254) -> ()
          n129 = case shown="\"IT Print\", 默认" w263 {
            tunnel: [0 1] -> w262
            frame "IT Print", Default {
            }
            frame "EE Print" {
            }
          }
          n130 = Decimal String To Number(string=w265) -> (number=w271:i32)  [unwired: 2 in, 1 out]
          n131 = To Upper Case(1:w285) -> (0:w292:string)
          n132 = To Upper Case(1:w279) -> (0:w282:string)
          n133 = To Upper Case(1:w283) -> (0:w287:string)
          n134 = To Upper Case(1:w301) -> (0:w306:string)
          n135 = local write "Port Type"(w271) -> ()
          n136 = To Upper Case(1:w300) -> (0:w303:string)
          n137 = Equal?(x=w292, y="TRUE") -> (x = y?=w290:bool)
          n138 = Equal?(x=w282, y="TRUE") -> (x = y?=w280:bool)
          n139 = Equal?(x=w287, y="TRUE") -> (x = y?=w286:bool)
          n140 = property on="VNA VISA" class="VISAName"("Value"=w276) -> ()  [unwired: 2 in, 2 out]
          n141 = Equal?(x=w306, y="TRUE") -> ()  [unwired: 1 out]
          n142 = Equal?(x=w303, y="TRUE") -> (x = y?=w302:bool)
          n143 = local write "打印模式"(w262) -> ()
          n144 = case shown="\"N5230A(C)\"" w314 {
            tunnel: [0 1 2] -> w313
            frame "E5071C", Default {
            }
            frame "N5230A(C)" {
            }
            frame "N5224A" {
            }
          }
          n145 = case shown="\"Dev3\"" w310 {
            tunnel: [0 1 2] -> w311
            frame "Dev1", Default {
            }
            frame "Dev2" {
            }
            frame "Dev3" {
            }
          }
          n146 = case shown="\"NI PCI-6509\", 默认" w312 {
            tunnel: [0 1] -> w266
            frame "NI PCI-6509", Default {
            }
            frame "LX MCU" {
            }
          }
          n147 = local write "Crosstalk  by Trace"(w290) -> ()
          n148 = local write "Local Database"(w302) -> ()
          n149 = local write "Dem 2X"(w286) -> ()
          n150 = local write "By Channel?"(w280) -> ()
          n151 = case shown="\"RS232 - IIC\", 默认" w260 {
            tunnel: [0 1] -> w261
            frame "RS232 - IIC", Default {
            }
            frame "LUXSHARE - IIC" {
            }
          }
          n152 = To Upper Case(1:w272) -> (0:w274:string)
          n153 = local write "RS232 I2C VISA"(w277) -> ()
          n154 = local write "VNA Model:"(w313) -> ()
          n155 = local write "Printer VISA"(w278) -> ()
          n156 = local write "DAQ  Model:"(w266) -> ()
          n157 = local write "DAQ Device"(w311) -> ()
          n158 = Equal?(x=w274, y="TRUE") -> (x = y?=w273:bool)
          n159 = local write "VISA COM"(w309) -> ()
          n160 = To Upper Case(1:w293) -> (0:w299:string)
          n161 = To Upper Case(1:w289) -> (0:w296:string)
          n162 = Equal?(x=w299, y="TRUE") -> (x = y?=w295:bool)
          n163 = Equal?(x=w296, y="TRUE") -> (x = y?=w294:bool)
          n164 = local write "upload"(w273) -> ()
          n165 = local write "Demo"(w295) -> ()
          n166 = local write "Manual"(w294) -> ()
          n167 = local write "Adaptor:"(w261) -> ()
          n168 = case shown="1" w266 {
            tunnel: [2 0] -> w268
            tunnel: [0 2] -> w267
            frame 0, Default {
            }
            frame 1 {
            }
          }
          n169 = disable-structure shown="禁用" {
            disable-tunnel: w273 -> [w317 _]
            frame Disabled {
              w318 = "Data UpLoad" ("项标识符")
              n170 = Current VI's Menubar() -> (w321:refnum<k9>)
              n171 = Get Menu Item Info(7:w318, 11:w321) -> (2:w319:string, 3:w320:refnum<k9>)  [unwired: 1 in, 5 out]
              n172 = Set Menu Item Info(6:w317, 7:w318, 9:TRUE ("已启用"), 10:w319, 11:w320) -> ()  [unwired: 2 in, 2 out]
            }
            frame Enabled {
            }
          }
          n173 = To Upper Case(1:w256) -> (0:w258:string)
          n174 = Equal?(x=w258, y="TRUE") -> (x = y?=w255:bool)
          n175 = property on="DAQ Device" class="Ring (严格)"("DisabledEnum"=w267) -> ()  [unwired: 2 in, 2 out]
          n176 = property on="VISA COM" class="VISAName"("DisabledEnum"=w268) -> ()  [unwired: 2 in, 2 out]
          n177 = local write "Use Counts?"(w255) -> ()
        }
        frame True {
          n178 = call-poly <vilib>:"Read From Spreadsheet File.vi"("file path (dialog if empty)"=w353) -> ("all rows"=w399:string[][])  [unwired: 6 in, 4 out]
          n179 = Index Array(array=w399, index (col)=1 ("禁用的索引 (列)")) -> (element=w397:string[])  [unwired: 1 in]
          n180 = Index Array(array=w397, index #1=0 ("索引"), index #6=5 ("索引"), index #11=10 ("索引"), index #16=15 ("索引")) -> (element #1=w359:string, element #2=w396:string, element #3=w394:string, element #4=w392:string, element #5=w391:string, element #6=w383:string, element #7=w382:string, element #8=w375:string, element #9=w371:string, element #10=w367:string, element #11=w365:string, element #12=w361:string, element #13=w343:string, element #14=w360:string, element #15=w355:string, element #16=w348:string, element #17=w345:string, element #18=w344:string, element #19=w339:string, element #20=w338:string)  [unwired: 16 in]
          n181 = local write "RS232 I2C Counts"(w338) -> ()
          n182 = case shown="\"IT Print\", 默认" w345 {
            tunnel: [0 1] -> w347
            frame "IT Print", Default {
            }
            frame "EE Print" {
            }
          }
          n183 = Decimal String To Number(string=w348) -> (number=w354:i32)  [unwired: 2 in, 1 out]
          n184 = local write "Port Type"(w354) -> ()
          n185 = To Upper Case(1:w367) -> (0:w374:string)
          n186 = To Upper Case(1:w361) -> (0:w364:string)
          n187 = To Upper Case(1:w365) -> (0:w369:string)
          n188 = To Upper Case(1:w383) -> (0:w388:string)
          n189 = To Upper Case(1:w382) -> (0:w385:string)
          n190 = Equal?(x=w374, y="TRUE") -> (x = y?=w372:bool)
          n191 = Equal?(x=w364, y="TRUE") -> (x = y?=w362:bool)
          n192 = Equal?(x=w369, y="TRUE") -> (x = y?=w368:bool)
          n193 = property on="VNA VISA" class="VISAName"("Value"=w359) -> ()  [unwired: 2 in, 2 out]